vi "Trajectory Builder.vi"() -> ()   [LabVIEW 2023] (continued)
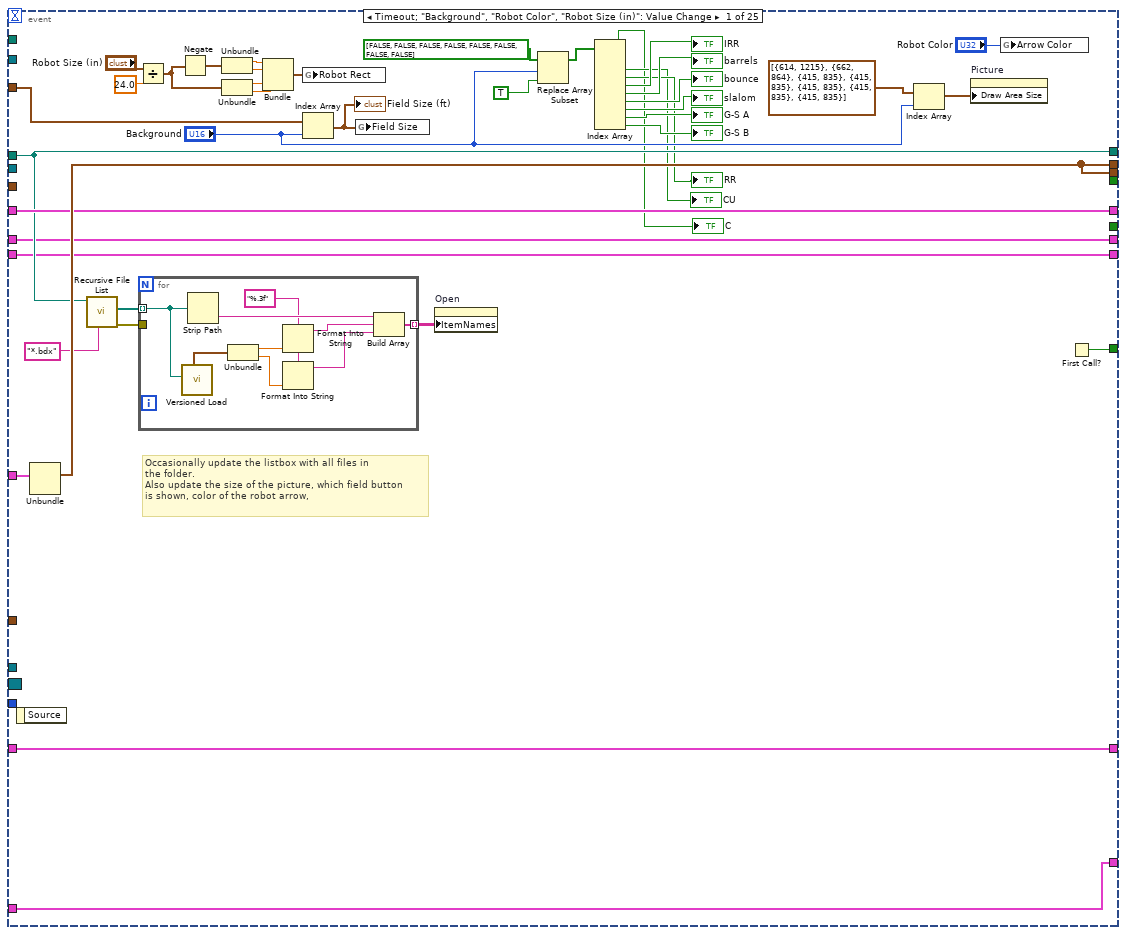
[diagram p3: hidden frame]
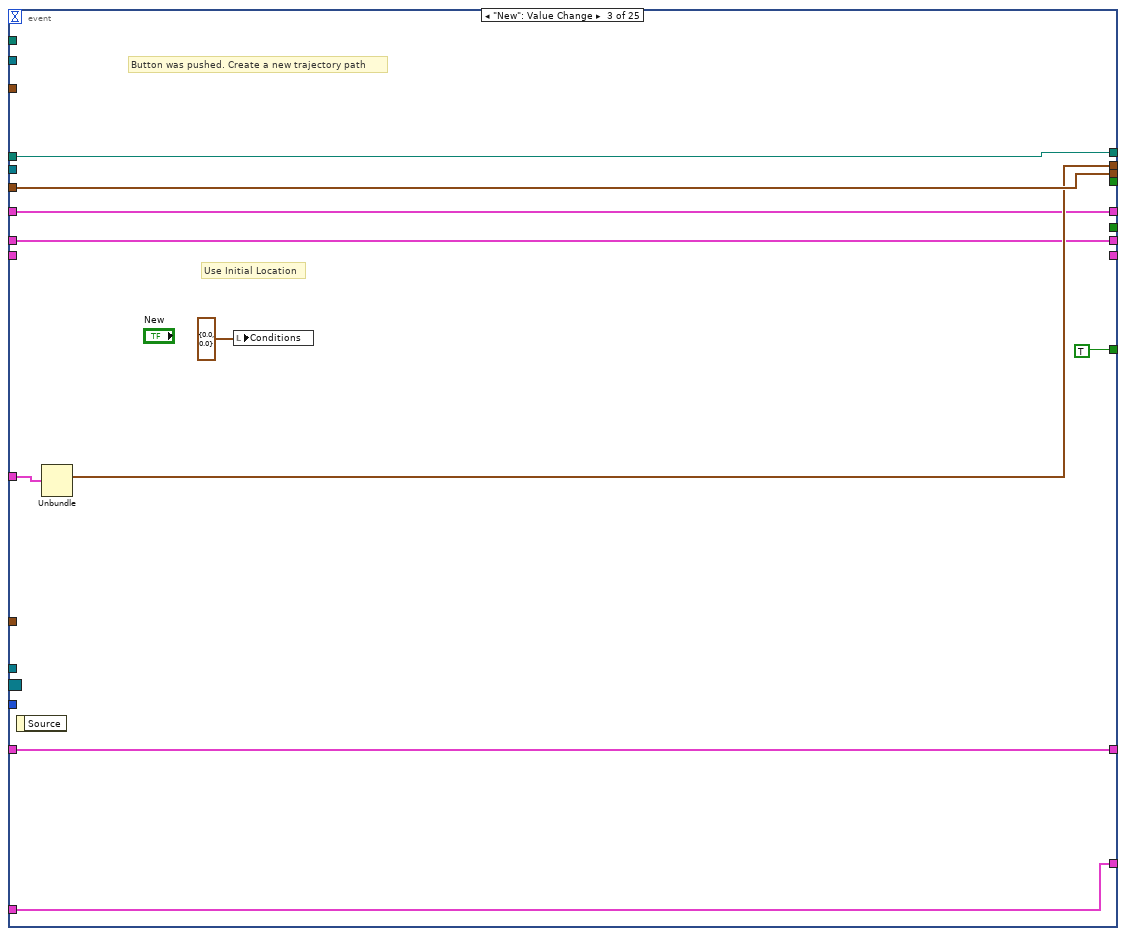
[diagram p4: hidden frame]
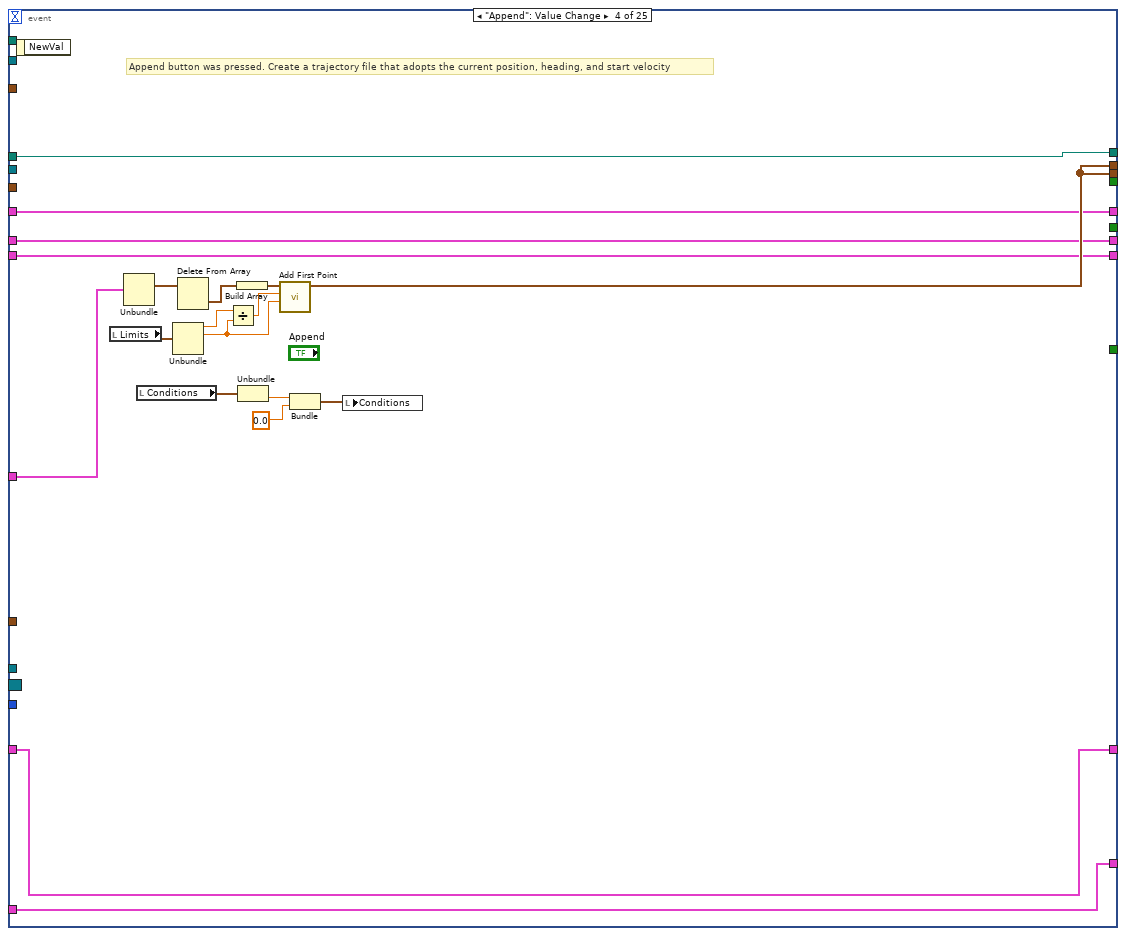
[diagram p5: hidden frame]
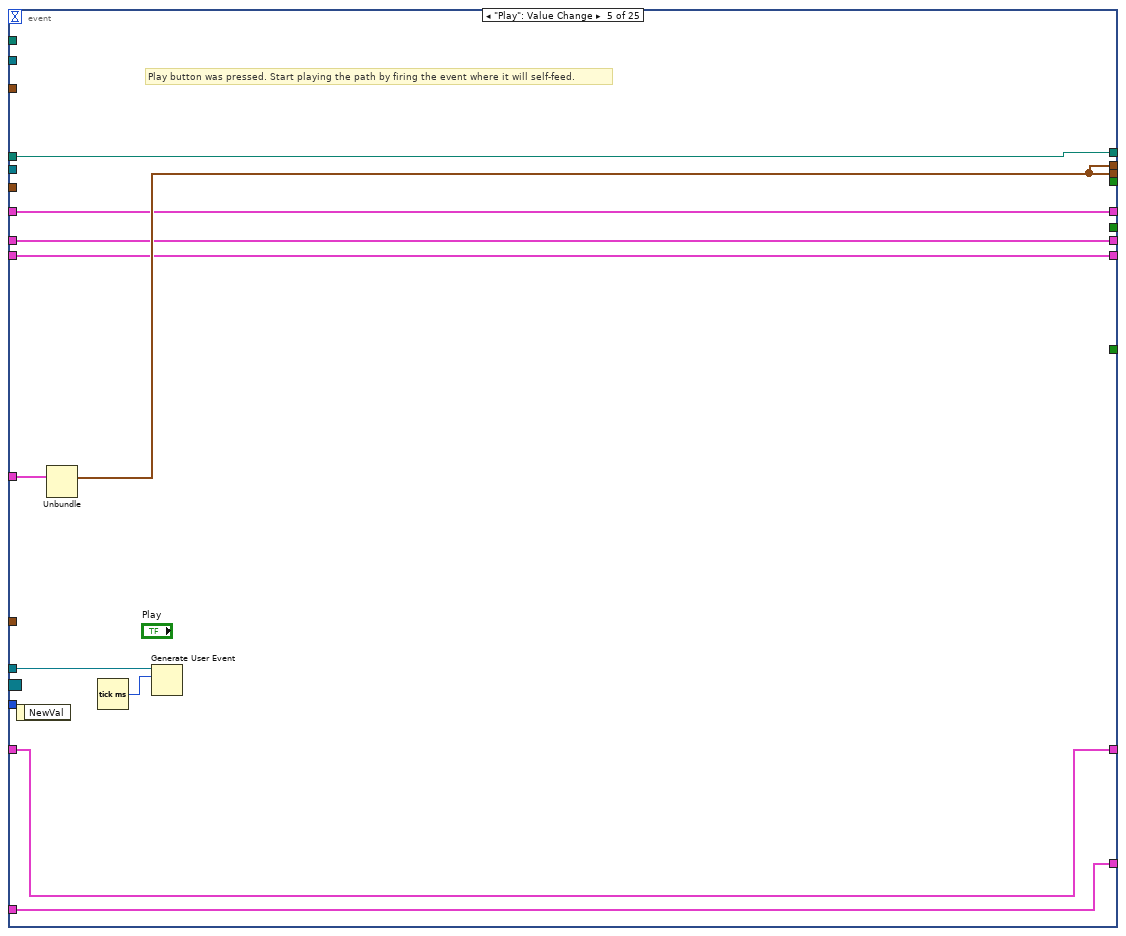
[diagram p6: hidden frame]
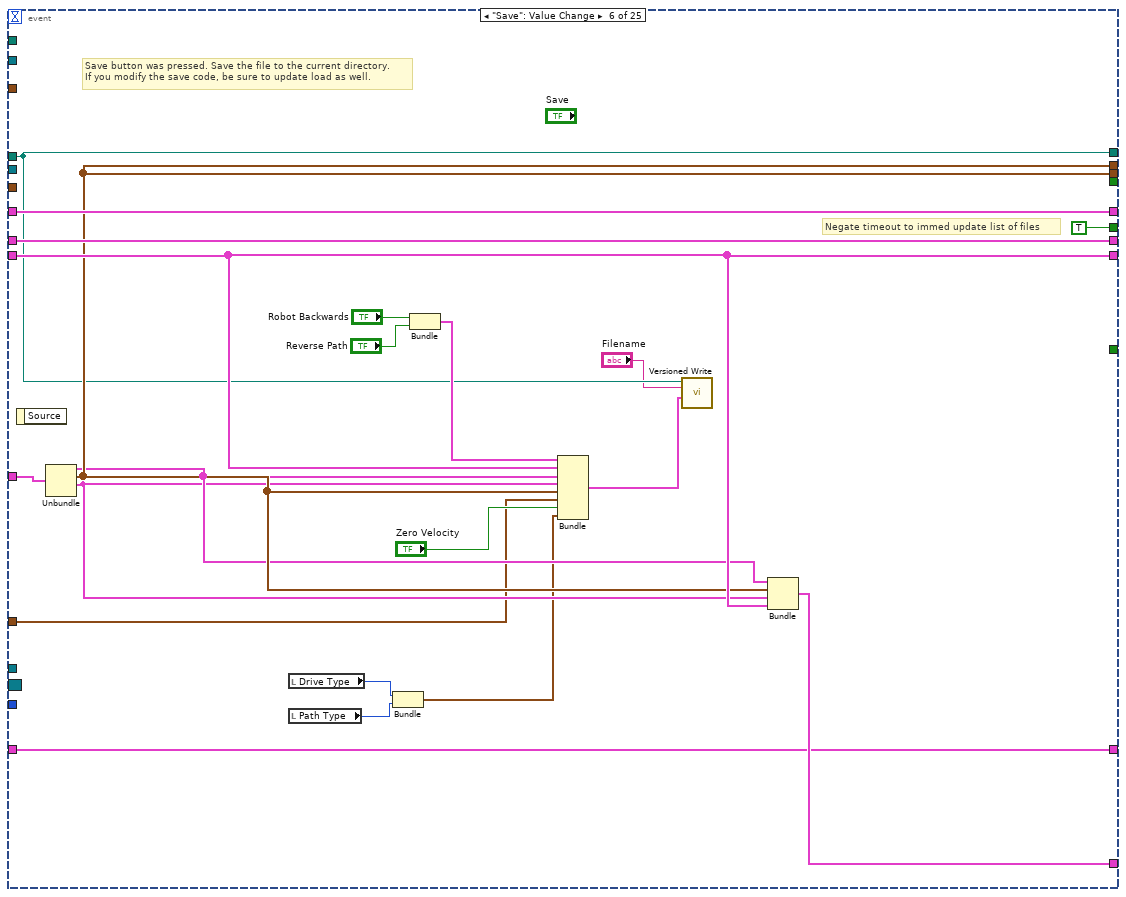
[diagram p7: hidden frame]
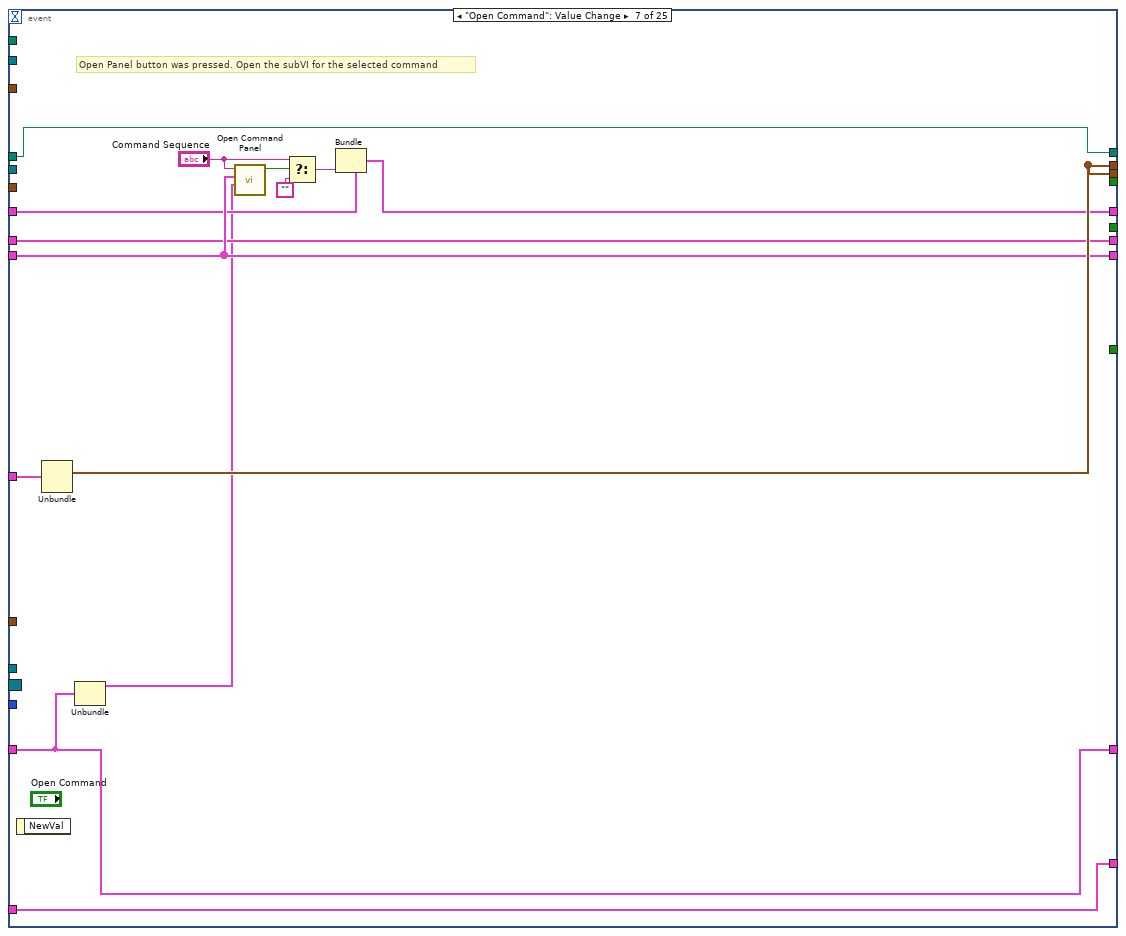
[diagram p8: hidden frame]
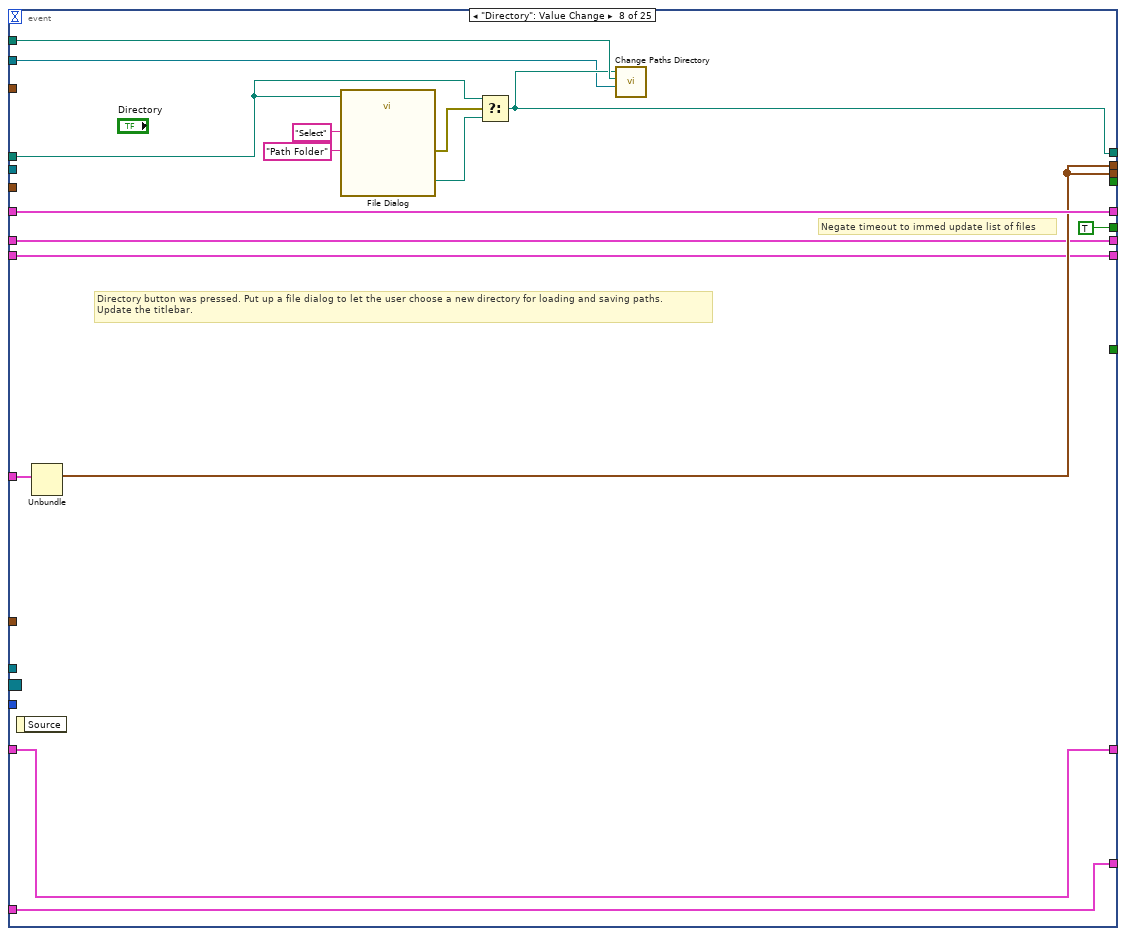
[diagram p9: hidden frame]
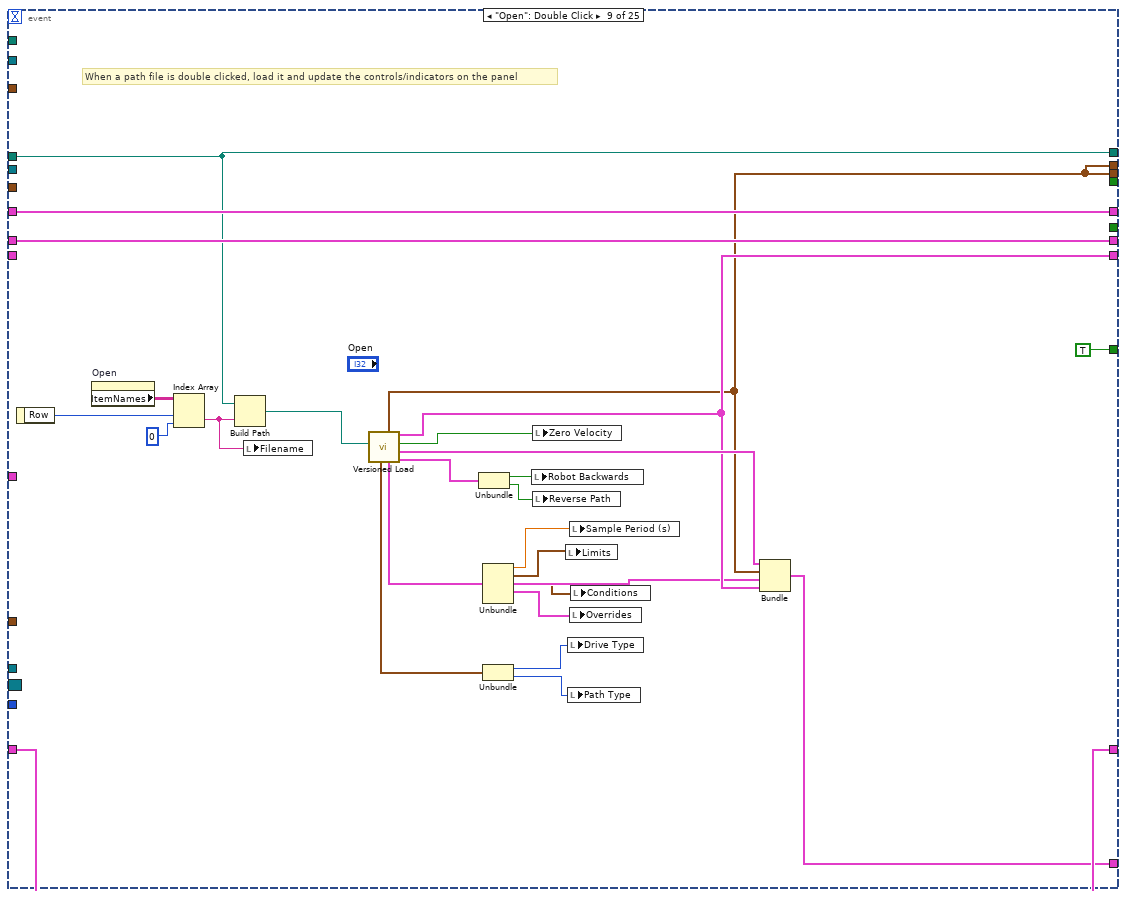
[diagram p10: hidden frame]
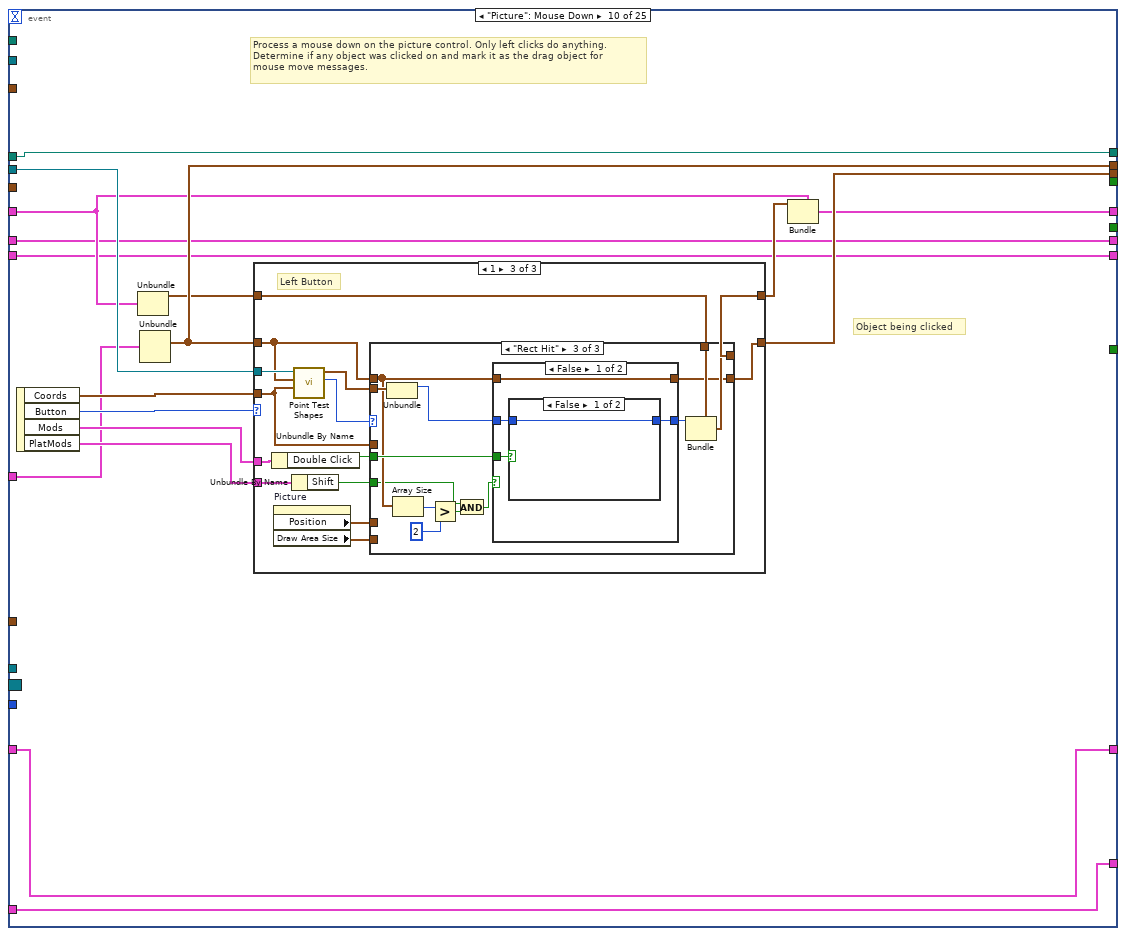
[diagram p11: hidden frame]
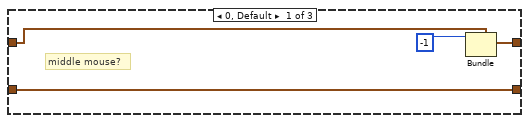
[diagram p12: hidden frame]
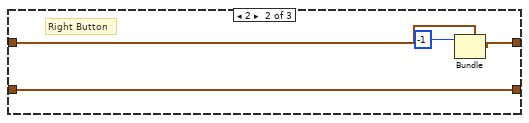
[diagram p13: hidden frame]
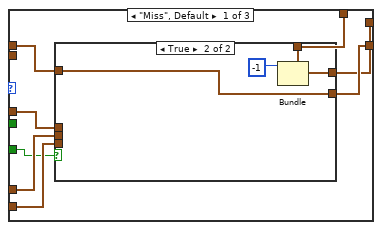
[diagram p14: hidden frame]
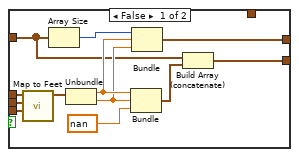
[diagram p15: hidden frame]
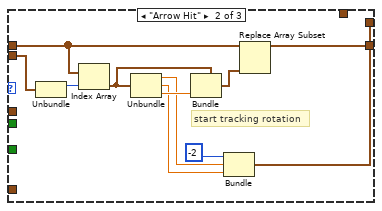
[diagram p16: hidden frame]
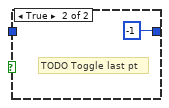
[diagram p17: hidden frame]
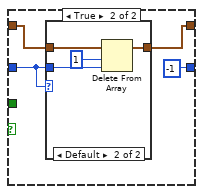
[diagram p18: hidden frame]
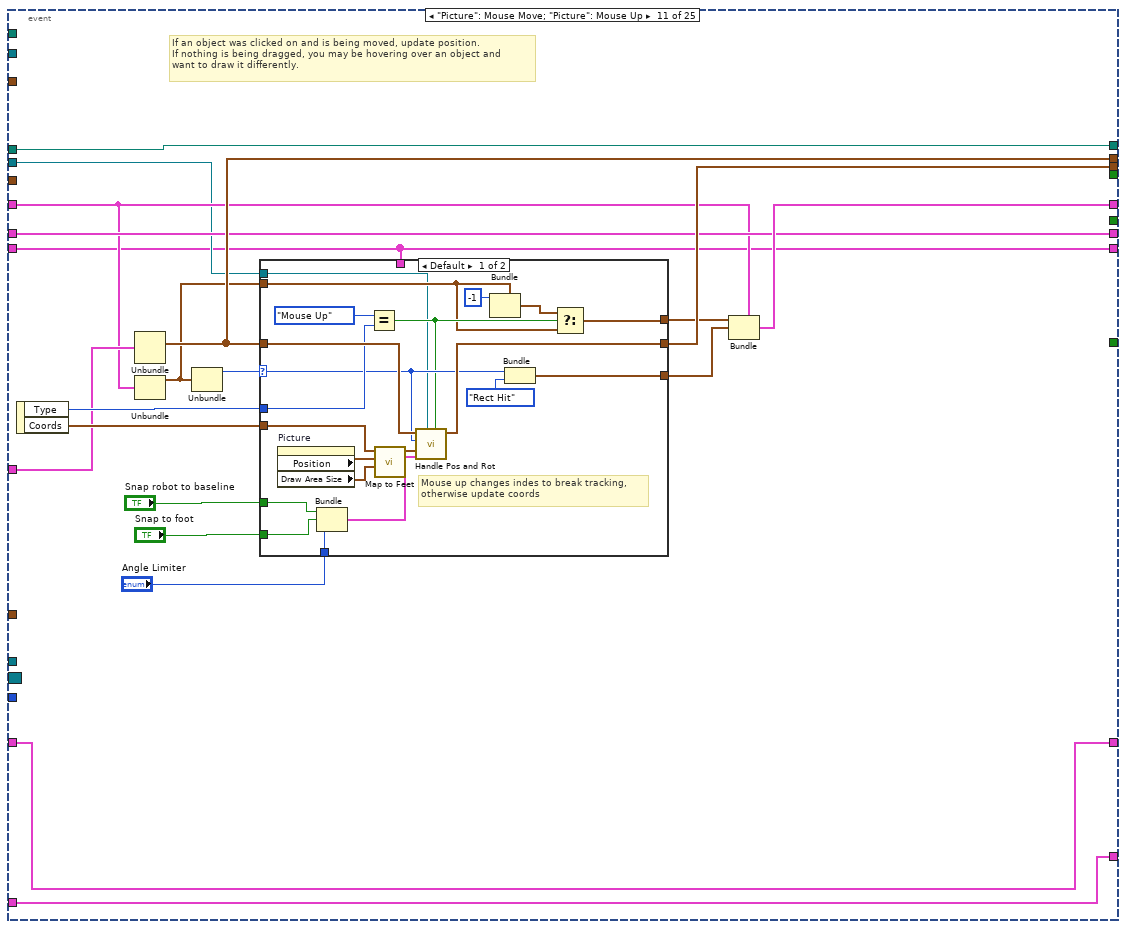
[diagram p20: hidden frame]
              tunnel: w827 -> [_ w834]
              tunnel: w822 -> [_ w830]
              tunnel: w821 -> [_ w835]
              frame False {
              }
              frame True {
                n322 = Bundle(cluster=w835, "Time (s)"=w834) -> (w831:cluster{"Time (s)":dbl, T2, bool})  [unwired: 2 in]
                n323 = Replace Array Subset(array=w832, new element=w831, index=w830) -> (w833:cluster{"Time (s)":dbl, T2, bool}[])
              }
            }
          }
        }
        n324 = event-data("Discard?"=w799) -> ()  [unwired: 1 in, 1 out]
        n325 = Not(x=w799) -> (.not. x?=w800:bool)
      }
      event "Command Palette": Mouse Move {
        # "Draw the hilite for the row that the mouse is over"
        n326 = event-data() -> ("Coords"=w843:T31)  [unwired: 1 in]
        n327 = Unbundle(w846) -> ("Updated Waypoints"=w845:cluster{"x":dbl, "y":dbl, "th":dbl}[])  [unwired: 3 out]
        n328 = control-ref of="Command Palette"() -> (w839:refnum<vi>)
        n329 = call "Picture Coord to Row.vi"("Row Height"=w838, "Coords"=w843, "Picture in"=w839) -> ("Row Index"=w840:i32, "Clicked in canvas"=w842:bool)  [unwired: 7 in]
        n330 = Unbundle(w836) -> ("Filtered Command Info Out"=w841:T1, "2D Picture"=w844:picture)  [unwired: 1 out]
        n331 = case shown="True" w842 {
          tunnel: w844 -> [_ w854]
          tunnel: w841 -> [_ _]
          tunnel: w838 -> [_ w852]
          tunnel: w840 -> [_ w851]
          frame False {
          }
          frame True {
            n332 = Multiply(x=w851, y=w852) -> (x*y=w857:i32)
            n333 = Add(x=w857, y=w852) -> (x+y=w858:i32)
            n334 = Bundle(0, w857, 300, w858) -> (w859:cluster{i32, i32, i32, i32})  [unwired: 1 in]
            n335 = call <vilib>:"Draw Rectangle.vi"("rect"=w859, "fill?(F)"=TRUE, "color(black)"=u32 10539263) -> ("new picture"=w861:picture)  [unwired: 6 in]
            n336 = Concatenate Strings(w861, w854) -> (→"Command Palette":picture)
          }
        }
      }
      event "Command Palette": Mouse Down {
        # "When a double click occurs in the command palette,\nadd the command to the command list at time T."
        n337 = event-data() -> ("Coords"=w873:T31, "Mods"=w875:cluster{"Double Click":bool, "Menu Key":bool})  [unwired: 1 in, 1 out]
        n338 = control-ref of="Command Palette"() -> (w874:refnum<vi>)
        n339 = Unbundle(w877) -> ("Updated Waypoints"=w876:cluster{"x":dbl, "y":dbl, "th":dbl}[])  [unwired: 3 out]
        n340 = call "Picture Coord to Row.vi"("Row Height"=w872, "Coords"=w873, "Picture in"=w874) -> ("Row Index"=w868:i32, "Clicked in canvas"=w871:bool)  [unwired: 7 in]
        n341 = Unbundle(w875) -> ("Double Click"=w870:bool)  [unwired: 1 out]
        n342 = Unbundle(w863) -> ("Filtered Command Info Out"=w867:T1)  [unwired: 2 out]
        n343 = Compound Arithmetic op=AND(w871, w870) -> (w869:bool)
        n344 = case shown="True" w869 {
          tunnel: w868 -> [_ w890]
          tunnel: w867 -> [_ w891]
          tunnel: w865 -> [w882 w886]
          tunnel: [w882 w883] -> w866
          frame False {
          }
          frame True {
            n345 = local read "Time (s)"() -> (w887:dbl)
            n346 = Index Array(array=w891, index=w890) -> (element=w889:T2)
            n347 = for {
              tunnel: w886 -> [w896] mode=indexing
              tunnel: w887 -> [w894]
              tunnel: [w892] -> w884
              i -> [w892]
              stop <- w893 stop-if-true
              n348 = Unbundle(w896) -> ("Time (s)"=w895:dbl)  [unwired: 2 out]
              n349 = Greater Or Equal?(x=w895, y=w894) -> (x >= y?=w893:bool)
            }
            n350 = Bundle("Time (s)"=w887, w889, TRUE) -> (w885:cluster{"Time (s)":dbl, T2, bool})  [unwired: 1 in]
            n351 = Insert Into Array(array=w886, index=w884, new element=w885) -> (w883:cluster{"Time (s)":dbl, T2, bool}[])
          }
        }
      }
    }
    n352 = feedback-in #1(w95) -> ()
    n353 = Unbundle(w70) -> (w69:T14)  [unwired: 3 out]
    n354 = Unbundle(w69) -> ("Limits"=w71:T11)  [unwired: 4 out]
    n355 = Unbundle(w71) -> ("Velocity (fps)"=w68:dbl)  [unwired: 3 out]
    n356 = flat-sequence {
      tunnel: ["Time (s)"] -> w110
      tunnel: ["Sample Period (s)"] -> w83
      tunnel: ["Limits"] -> w62
      tunnel: ["Conditions"] -> w48
      tunnel: [w125] -> w72
      tunnel: ["Overrides"] -> w47
      tunnel: w76 -> [w125]
      tunnel: w75 -> [w127]
      tunnel: ["Hide Path"] -> w66
      tunnel: ["Stoopid Overlap %"] -> w65
      tunnel: ["Angular Limits"] -> w46
      tunnel: [w119] -> w43
      frame #0 {
        n357 = control-ref of="Command Sequence"() -> (w128:refnum<vi>)
        n358 = global write "Global Settings.vi" "> 90?"("Allow Angles > 90") -> ()
        n359 = global write "Global Settings.vi" "Turn Angle Limit (deg)"("Turn Angle Limit (deg)") -> ()
        n360 = call "Format Tree.vi"("Update"=w127, "Commands"=w125, "Tree Refnum"=w128) -> ()  [unwired: 9 in]
        n361 = local read "Overrides"() -> (w119:T10)
      }
    }
    n362 = Unbundle(w62) -> ("Accel (fps^2)"=w61:dbl)  [unwired: 3 out]
    n363 = Divide(x=w110, y=w83) -> (x/y=w103:dbl)
    n364 = Bundle("Sample Period (s)"=w83, "Limits"=w62, "Conditions"=w48, "Overrides"=w47, "Angular Limits"=w46) -> (w63:T14)  [unwired: 1 in]
    n365 = call "Enforce Robot Rules.vi"("max V"=w68, "Drive Type"="Drive Type", "Overrides"=w43, "turn accel"=w61, "Disable"=w56, "New Points"=w105, "Original Points"=w104) -> ("Overrides Out"=w49:T10, "Points out"=w45:cluster{"x":dbl, "y":dbl, "th":dbl}[])  [unwired: 3 in]
    n366 = call "GenNewTraj.vi"("Drive Type"="Drive Type", "Stoopid Overlap %"=w65, "Path Type"="Path Type", "Parameters"=w63, "Points in"=w45) -> ("Time & Dist"=w55:cluster{"Time (s)":dbl, "Distance (ft)":dbl}, "Valid"=w84:bool, "Trajectory Data"=w92:T5, "Updated Waypoints"=w96:cluster{"x":dbl, "y":dbl, "th":dbl}[])  [unwired: 3 in]
    "Trajectory Data" <- w92
    n367 = local write "WayPoints"(w45) -> ()
    n368 = local write "Overrides"(w49) -> ()
    n369 = Unbundle(w55) -> ("Time (s)"=w53:dbl, "Distance (ft)"=→"Distance (ft)":dbl)
    "Duration (s)" <- w53
    n370 = Unbundle(w90) -> ("Hover Object"=w89:T17)  [unwired: 2 out]
    n371 = Bundle(cluster=T20 {"Trajectory Data"=[], "Updated Waypoints"=[], {"Sample Period (s)"=0.0, "Limits"={"Velocity (fps)"=0.0, "Accel (fps^2)"=0.0, "Jerk (fps^3)"=0.0, "StoopidFast (fps)"=0.0}, "Conditions"={"vInitial (fps)"=0.0, "vFinal (fps)"=0.0}, "Overrides"=[], "Angular Limits"={"Velocity (deg/s)"=6.0, "Accel (deg/s^2)"=15.0, "Jerk (deg/s^3)"=150.0}}, "Commands out"=[]} ("output cluster"), "Trajectory Data"=w92, "Updated Waypoints"=w96, w63, "Commands out"=w72) -> (w50:T20)
    n372 = property on="Time (s)" class="Slide (strict)"("Scale.Minimum"=0.0 ("Scale.Range:Minimum"), "Scale.Maximum"=w53) -> ()  [unwired: 2 in, 2 out]
    n373 = call "Draw Trajectory.vi"("Robot Index"=w103, "Hide Path"=w66, "new picture in"=picture data[5B] ("new picture"), "Trajectory Data"=w92, "Picture in"=w113) -> ("Path Points"=w97:cluster{"x":dbl, "y":dbl}[], "Output Point"=w109:T38, "new picture"=w111:picture)  [unwired: 4 in]
    n374 = call "Draw Shapes.vi"("Path Points"=w97, "Sample Period (s)"=w83, "Output Point"=w109, "Commands"=w72, "Results"=w89, "new picture in"=w111, "Points"=w96, "Picture in"=w113) -> ("new picture out"=→"Picture":picture)  [unwired: 3 in]
    n375 = call "Update Annotations.vi"("Sample Period"=w83, "Commands"=w72, "Trajectory Data"=w92, "Robot Pt Index"=w103) -> ("Redraw"=w74:bool, "Velocity Trace"=w73:dbl[], "Annotation Data"=w102:T39)  [unwired: 5 in]
    n376 = case shown="True" w74 {
      tunnel: w102 -> [_ w898]
      tunnel: w73 -> [_ w897]
      frame False {
      }
      frame True {
        n377 = property on="fps" class="WFGraph (strict)"("AnntList"=w898) -> ()  [unwired: 2 in, 2 out]
        "fps" <- w897
      }
    }
    n378 = disable-structure shown="Disabled" {
      disable-tunnel: w84 -> [w116 _]
      frame Disabled {
        n379 = Select(t=cluster{u32, u32}[] [{14869218, 14869218}] ("Colors [4]"), s=w116, f=cluster{u32, u32}[] [{6094681, 6094681}] ("Colors [4]")) -> ()  [unwired: 1 out]
      }
      frame Enabled {
      }
    }
    n380 = control-ref of="Save"() -> (w59:refnum<vi>)
    n381 = Select(t=0, s=w85, f=2000) -> (s? t:f=w86:i32)
    n382 = call "Saved Checker.vi"("comp B"=w98, "comp A"=w50, "Save button ref"=w59) -> ()  [unwired: 1 in]
  }
  n383 = local write "Time (s)"(0.0 ("Time")) -> ()
